vi "Dresden R2R Sputter 03.02.2018 IY24.vi"() -> ()   [LabVIEW 2009] (continued)
                              }
                              frame #1 {
                              }
                            }
                          }
                        }
                      }
                      frame #1 {
                      }
                    }
                  }
                  frame #1 {
                  }
                }
              }
              frame #1 {
              }
            }
          }
          frame #3 {
            # "STARTED UP CH2"
            n11092 = disable-structure shown="Disabled" {
              frame #0 {
                n11093 = local read "Semi"() -> (w17910:bool)
                n11094 = case shown="False" w17910 {
                  frame #0 {
                    n11095 = local read "started_up_ch2"() -> (w17911:bool)
                    n11096 = case shown="False" w17911 {
                      frame #0 {
                        n11097 = stacked-sequence {
                          frame #0 {
                            n11098 = local read "Semi"() -> (w17912:bool)
                            n11099 = case shown="False" w17912 {
                              frame #0 {
                                n11100 = local write "Start_up_ch2"(TRUE ("Start_up_ch2")) -> ()
                              }
                              frame #1 {
                              }
                            }
                          }
                          frame #1 {
                            n11101 = local read "Semi"() -> (w17914:bool)
                            n11102 = case shown="False" w17914 {
                              frame #0 {
                                n11103 = Wait (ms)(milliseconds to wait=u32 18000) -> ()  [unwired: 1 out]
                              }
                              frame #1 {
                              }
                            }
                          }
                          frame #2 {
                            n11104 = local read "Semi"() -> (w17916:bool)
                            n11105 = case shown="False" w17916 {
                              frame #0 {
                                n11106 = while {
                                i -> [w17921]
                                stop <- w17918 stop-if-true
                                n11107 = Greater?(x=w17921, y=90) -> (0:w17919:bool)
                                n11108 = local read "started_up_ch2"() -> (w17917:bool)
                                n11109 = case shown="True" w17919 {
                                frame #0 {
                                }
                                frame #1 {
                                n11110 = local write "Semi"(TRUE ("Semi")) -> ()
                                n11111 = local write "Error Message"("Chamber 2 Pressure is not suitable  \nfor transfer process!\nPlease check connections." ("Error Message")) -> ()
                                }
                                }
                                n11112 = case shown="False" w17917 {
                                tunnel: [FALSE TRUE] -> w17918
                                frame #0 {
                                n11113 = Wait Until Next ms Multiple(millisecond multiple=u32 200) -> ()  [unwired: 1 out]
                                }
                                frame #1 {
                                }
                                }
                                }
                              }
                              frame #1 {
                              }
                            }
                          }
                          frame #3 {
                            n11114 = local read "Semi"() -> (w17927:bool)
                            n11115 = case shown="False" w17927 {
                              frame #0 {
                                n11116 = local write "CH1_2_trns_1"(TRUE ("CH1_2_trns_0")) -> ()
                                n11117 = Wait (ms)(milliseconds to wait=u32 1000) -> ()  [unwired: 1 out]
                              }
                              frame #1 {
                              }
                            }
                          }
                        }
                      }
                      frame #1 {
                      }
                    }
                  }
                  frame #1 {
                  }
                }
              }
              frame #1 {
              }
            }
          }
          frame #4 {
            # "TRNS GV OPEN"
            n11118 = local read "Semi"() -> (w17930:bool)
            n11119 = case shown="False" w17930 {
              frame #0 {
                n11120 = stacked-sequence {
                  frame #0 {
                    n11121 = local read "Semi"() -> (w17931:bool)
                    n11122 = case shown="False" w17931 {
                      frame #0 {
                        n11123 = while {
                          i -> [w17938]
                          stop <- w17933 stop-if-true
                          n11124 = Greater?(x=w17938, y=50) -> (0:w17936:bool)
                          n11125 = local read "Ch1_Trns_gv_bp2_di"() -> (w17932:bool)
                          n11126 = case shown="True" w17936 {
                            frame #0 {
                            }
                            frame #1 {
                              n11127 = local write "Semi"(TRUE ("Semi")) -> ()
                              n11128 = local write "Error Message"("Transfer process was cancelled.\nPlease check CH1-Trns-GV connections." ("Error Message")) -> ()
                            }
                          }
                          n11129 = case shown="False" w17932 {
                            tunnel: [FALSE TRUE] -> w17935
                            frame #0 {
                              n11130 = Wait Until Next ms Multiple(millisecond multiple=u32 200) -> ()  [unwired: 1 out]
                              n11131 = local write "Ch1_Trns_gv_bp2_do"(TRUE ("Ch1_pet_cool_up_do")) -> ()
                            }
                            frame #1 {
                            }
                          }
                          n11132 = local read "Semi"() -> (w17934:bool)
                          n11133 = Or(x=w17935, y=w17934) -> (x .or. y?=w17933:bool)
                        }
                      }
                      frame #1 {
                      }
                    }
                  }
                  frame #1 {
                    n11134 = local read "Semi"() -> (w17945:bool)
                    n11135 = case shown="False" w17945 {
                      frame #0 {
                        n11136 = Wait (ms)(milliseconds to wait=u32 500) -> ()  [unwired: 1 out]
                      }
                      frame #1 {
                      }
                    }
                  }
                  frame #2 {
                    n11137 = local read "Semi"() -> (w17947:bool)
                    n11138 = case shown="False" w17947 {
                      frame #0 {
                        n11139 = while {
                          i -> [w17954]
                          stop <- w17949 stop-if-true
                          n11140 = Greater?(x=w17954, y=50) -> (0:w17952:bool)
                          n11141 = local read "Ch2_trns_gv_bp_di"() -> (w17948:bool)
                          n11142 = case shown="True" w17952 {
                            frame #0 {
                            }
                            frame #1 {
                              n11143 = local write "Semi"(TRUE ("Semi")) -> ()
                              n11144 = local write "Error Message"("Transfer process was cancelled.\nPlease check CH1-Trns-GV connections." ("Error Message")) -> ()
                            }
                          }
                          n11145 = case shown="False" w17948 {
                            tunnel: [FALSE TRUE] -> w17951
                            frame #0 {
                              n11146 = Wait Until Next ms Multiple(millisecond multiple=u32 200) -> ()  [unwired: 1 out]
                              n11147 = local write "Ch2_trns_gv_bp_do"(TRUE ("Ch1_pet_cool_up_do")) -> ()
                            }
                            frame #1 {
                            }
                          }
                          n11148 = local read "Semi"() -> (w17950:bool)
                          n11149 = Or(x=w17951, y=w17950) -> (x .or. y?=w17949:bool)
                        }
                      }
                      frame #1 {
                      }
                    }
                  }
                  frame #3 {
                    n11150 = local read "Semi"() -> (w17961:bool)
                    n11151 = case shown="False" w17961 {
                      frame #0 {
                        n11152 = Wait (ms)(milliseconds to wait=u32 500) -> ()  [unwired: 1 out]
                      }
                      frame #1 {
                      }
                    }
                  }
                }
              }
              frame #1 {
              }
            }
          }
          frame #5 {
            # "TRNS GV OPEN"
            n11153 = local read "Semi"() -> (w17963:bool)
            n11154 = case shown="False" w17963 {
              frame #0 {
                n11155 = stacked-sequence {
                  frame #0 {
                    n11156 = local read "Semi"() -> (w17964:bool)
                    n11157 = case shown="False" w17964 {
                      frame #0 {
                        n11158 = local write "Ch1_Trns_gv_close_do"(FALSE ("Ch1_pet_cool_up_do")) -> ()
                      }
                      frame #1 {
                      }
                    }
                  }
                  frame #1 {
                    n11159 = local read "Semi"() -> (w17966:bool)
                    n11160 = case shown="False" w17966 {
                      frame #0 {
                        n11161 = while {
                          i -> [w17973]
                          stop <- w17968 stop-if-true
                          n11162 = Greater?(x=w17973, y=500) -> (0:w17971:bool)
                          n11163 = local read "Ch1_Trns_gv_open_di"() -> (w17967:bool)
                          n11164 = case shown="True" w17971 {
                            frame #0 {
                            }
                            frame #1 {
                              n11165 = local write "Semi"(TRUE ("Semi")) -> ()
                              n11166 = local write "Error Message"("Transfer process was cancelled.\nPlease check CH1-Trns-GV connections." ("Error Message")) -> ()
                            }
                          }
                          n11167 = case shown="False" w17967 {
                            tunnel: [FALSE TRUE] -> w17970
                            frame #0 {
                              n11168 = Wait Until Next ms Multiple(millisecond multiple=u32 200) -> ()  [unwired: 1 out]
                              n11169 = local write "Ch1_Trns_gv_open_do"(TRUE ("Ch1_pet_cool_up_do")) -> ()
                            }
                            frame #1 {
                            }
                          }
                          n11170 = local read "Semi"() -> (w17969:bool)
                          n11171 = Or(x=w17970, y=w17969) -> (x .or. y?=w17968:bool)
                        }
                      }
                      frame #1 {
                      }
                    }
                  }
                  frame #2 {
                    n11172 = local read "Semi"() -> (w17980:bool)
                    n11173 = case shown="False" w17980 {
                      frame #0 {
                        n11174 = local write "CH1_2trns_2"(TRUE ("CH1_2trns_5")) -> ()
                        n11175 = Wait (ms)(milliseconds to wait=u32 500) -> ()  [unwired: 1 out]
                      }
                      frame #1 {
                      }
                    }
                  }
                }
              }
              frame #1 {
              }
            }
          }
          frame #6 {
            # "TRNS GV control Trnsgv 2_3"
            n11176 = local read "Semi"() -> (w17983:bool)
            n11177 = case shown="False" w17983 {
              frame #0 {
                n11178 = stacked-sequence {
                  frame #0 {
                    n11179 = local read "Semi"() -> (w17984:bool)
                    n11180 = case shown="False" w17984 {
                      frame #0 {
                        n11181 = while {
                          i -> [w17991]
                          stop <- w17986 stop-if-true
                          n11182 = Greater?(x=w17991, y=50) -> (0:w17989:bool)
                          n11183 = local read "Ch1_TGV_control_di"() -> (w17985:bool)
                          n11184 = case shown="True" w17989 {
                            frame #0 {
                            }
                            frame #1 {
                              n11185 = local write "Semi"(TRUE ("Semi")) -> ()
                              n11186 = local write "Error Message"("Transfer process was cancelled.\nPlease check TRNS-GV connections." ("Error Message")) -> ()
                            }
                          }
                          n11187 = case shown="True" w17985 {
                            tunnel: [TRUE FALSE] -> w17988
                            frame #0 {
                            }
                            frame #1 {
                              n11188 = Wait Until Next ms Multiple(millisecond multiple=u32 200) -> ()  [unwired: 1 out]
                              n11189 = local write "Ch1_TGV_control_do"(FALSE ("Ch1_pet_cool_up_do")) -> ()
                            }
                          }
                          n11190 = local read "Semi"() -> (w17987:bool)
                          n11191 = Or(x=w17988, y=w17987) -> (x .or. y?=w17986:bool)
                        }
                      }
                      frame #1 {
                      }
                    }
                  }
                  frame #1 {
                    n11192 = local read "Semi"() -> (w17998:bool)
                    n11193 = case shown="False" w17998 {
                      frame #0 {
                        n11194 = local write "CH1_2trns_3"(TRUE ("CH1_2trns_5")) -> ()
                        n11195 = Wait (ms)(milliseconds to wait=u32 500) -> ()  [unwired: 1 out]
                      }
                      frame #1 {
                      }
                    }
                  }
                }
              }
              frame #1 {
              }
            }
          }
          frame #7 {
            # "TRNS GV control Trnsgv 2_3"
            n11196 = local read "Semi"() -> (w18001:bool)
            n11197 = case shown="False" w18001 {
              frame #0 {
                n11198 = stacked-sequence {
                  frame #0 {
                    n11199 = local read "Semi"() -> (w18002:bool)
                    n11200 = case shown="False" w18002 {
                      frame #0 {
                        n11201 = while {
                          i -> [w18009]
                          stop <- w18004 stop-if-true
                          n11202 = Greater?(x=w18009, y=50) -> (0:w18007:bool)
                          n11203 = local read "Ch2_Trns_interlock_di"() -> (w18003:bool)
                          n11204 = case shown="True" w18007 {
                            frame #0 {
                            }
                            frame #1 {
                              n11205 = local write "Semi"(TRUE ("Semi")) -> ()
                              n11206 = local write "Error Message"("Transfer process was cancelled.\nPlease check TRNS-GV connections." ("Error Message")) -> ()
                            }
                          }
                          n11207 = case shown="False" w18003 {
                            tunnel: [w18011 TRUE] -> w18006
                            frame #0 {
                              n11208 = local read "Ch2_TGV_control_di"() -> (w18010:bool)
                              n11209 = case shown="False" w18010 {
                                tunnel: [FALSE TRUE] -> w18011
                                frame #0 {
                                n11210 = Wait Until Next ms Multiple(millisecond multiple=u32 200) -> ()  [unwired: 1 out]
                                n11211 = local write "Ch2_TGV_control_do"(TRUE ("Ch1_pet_cool_up_do")) -> ()
                                }
                                frame #1 {
                                }
                              }
                            }
                            frame #1 {
                            }
                          }
                          n11212 = local read "Semi"() -> (w18005:bool)
                          n11213 = Or(x=w18006, y=w18005) -> (x .or. y?=w18004:bool)
                        }
                      }
                      frame #1 {
                      }
                    }
                  }
                  frame #1 {
                    n11214 = local read "Semi"() -> (w18019:bool)
                    n11215 = case shown="False" w18019 {
                      frame #0 {
                        n11216 = local write "CH1_2trns_3"(TRUE ("CH1_2trns_5")) -> ()
                        n11217 = Wait (ms)(milliseconds to wait=u32 500) -> ()  [unwired: 1 out]
                      }
                      frame #1 {
                      }
                    }
                  }
                }
              }
              frame #1 {
              }
            }
          }
          frame #8 {
            # "TRNS GV control Trnsgv 3_4"
            n11218 = local read "Semi"() -> (w18022:bool)
            n11219 = case shown="False" w18022 {
              frame #0 {
                n11220 = stacked-sequence {
                  frame #0 {
                    n11221 = local read "Semi"() -> (w18023:bool)
                    n11222 = case shown="False" w18023 {
                      frame #0 {
                        n11223 = while {
                          i -> [w18030]
                          stop <- w18025 stop-if-true
                          n11224 = Greater?(x=w18030, y=50) -> (0:w18028:bool)
                          n11225 = local read "Ch3_Trns_interlock_di"() -> (w18024:bool)
                          n11226 = case shown="True" w18028 {
                            frame #0 {
                            }
                            frame #1 {
                              n11227 = local write "Semi"(TRUE ("Semi")) -> ()
                              n11228 = local write "Error Message"("Transfer process was cancelled.\nPlease check TRNS-GV connections." ("Error Message")) -> ()
                            }
                          }
                          n11229 = case shown="False" w18024 {
                            tunnel: [w18032 TRUE] -> w18027
                            frame #0 {
                              n11230 = local read "Ch3_TGV_control_di"() -> (w18031:bool)
                              n11231 = case shown="False" w18031 {
                                tunnel: [FALSE TRUE] -> w18032
                                frame #0 {
                                n11232 = Wait Until Next ms Multiple(millisecond multiple=u32 200) -> ()  [unwired: 1 out]
                                n11233 = local write "Ch3_TGV_control_do"(TRUE ("Ch1_pet_cool_up_do")) -> ()
                                }
                                frame #1 {
                                }
                              }
                            }
                            frame #1 {
                            }
                          }
                          n11234 = local read "Semi"() -> (w18026:bool)
                          n11235 = Or(x=w18027, y=w18026) -> (x .or. y?=w18025:bool)
                        }
                      }
                      frame #1 {
                      }
                    }
                  }
                  frame #1 {
                    n11236 = local read "Semi"() -> (w18040:bool)
                    n11237 = case shown="False" w18040 {
                      frame #0 {
                        n11238 = local write "CH1_2trns_4"(TRUE ("CH1_2trns_5")) -> ()
                        n11239 = Wait (ms)(milliseconds to wait=u32 500) -> ()  [unwired: 1 out]
                      }
                      frame #1 {
                      }
                    }
                  }
                }
              }
              frame #1 {
              }
            }
          }
          frame #9 {
            # "Right slow deactive"
            n11240 = local read "Semi"() -> (w18043:bool)
            n11241 = case shown="False" w18043 {
              frame #0 {
                n11242 = stacked-sequence {
                  frame #0 {
                    n11243 = local read "Semi"() -> (w18044:bool)
                    n11244 = case shown="False" w18044 {
                      frame #0 {
                        n11245 = while {
                          i -> [w18047]
                          stop <- w18048 stop-if-true
                          n11246 = Greater?(x=w18047, y=50) -> (0:w18045:bool)
                          n11247 = local read "Cnt_Right_slow_di"() -> (w18051:bool)
                          n11248 = case shown="True" w18045 {
                            frame #0 {
                            }
                            frame #1 {
                              n11249 = local write "Semi"(TRUE ("Semi")) -> ()
                              n11250 = local write "Error Message"("Transfer process was\ncancelled.Please check right slow sensor." ("Error Message")) -> ()
                            }
                          }
                          n11251 = case shown="False" w18051 {
                            tunnel: [FALSE ("Ch1_pet_cool_up_do") TRUE ("Ch1_pet_cool_up_do")] -> w18050
                            frame #0 {
                              n11252 = Wait Until Next ms Multiple(millisecond multiple=u32 200) -> ()  [unwired: 1 out]
                              n11253 = local write "Cnt_Right_slow_do"(TRUE ("Ch1_pet_cool_up_do")) -> ()
                            }
                            frame #1 {
                            }
                          }
                          n11254 = local read "Semi"() -> (w18049:bool)
                          n11255 = Or(x=w18050, y=w18049) -> (x .or. y?=w18048:bool)
                        }
                      }
                      frame #1 {
                      }
                    }
                  }
                  frame #1 {
                    n11256 = local read "Semi"() -> (w18058:bool)
                    n11257 = case shown="False" w18058 {
                      frame #0 {
                        n11258 = local write "CH1_2trns_5"(TRUE ("CH1_2trns_7")) -> ()
                        n11259 = Wait (ms)(milliseconds to wait=u32 500) -> ()  [unwired: 1 out]
                      }
                      frame #1 {
                      }
                    }
                  }
                }
              }
              frame #1 {
              }
            }
          }
          frame #10 {
            # "Right limit deactive"
            n11260 = local read "Semi"() -> (w18061:bool)
            n11261 = case shown="False" w18061 {
              frame #0 {
                n11262 = stacked-sequence {
                  frame #0 {
                    n11263 = local read "Semi"() -> (w18062:bool)
                    n11264 = case shown="False" w18062 {
                      frame #0 {
                        n11265 = while {
                          i -> [w18063]
                          stop <- w18067 stop-if-true
                          n11266 = Greater?(x=w18063, y=50) -> (0:w18065:bool)
                          n11267 = local read "Cnt_Right_limit_di"() -> (w18069:bool)
                          n11268 = case shown="True" w18065 {
                            frame #0 {
                            }
                            frame #1 {
                              n11269 = local write "Semi"(TRUE ("Semi")) -> ()
                              n11270 = local write "Error Message"("Transfer process was\ncancelled.Please check right limit sensor." ("Error Message")) -> ()
                            }
                          }
                          n11271 = case shown="False" w18069 {
                            tunnel: [FALSE ("Ch1_pet_cool_up_do") TRUE ("Ch1_pet_cool_up_do")] -> w18068
                            frame #0 {
                              n11272 = Wait Until Next ms Multiple(millisecond multiple=u32 200) -> ()  [unwired: 1 out]
                              n11273 = local write "Cnt_Right_limit_do"(TRUE ("Ch1_pet_cool_up_do")) -> ()
                            }
                            frame #1 {
                            }
                          }
                          n11274 = local read "Semi"() -> (w18066:bool)
                          n11275 = Or(x=w18068, y=w18066) -> (x .or. y?=w18067:bool)
                        }
                      }
                      frame #1 {
                      }
                    }
                  }
                  frame #1 {
                    n11276 = local read "Semi"() -> (w18076:bool)
                    n11277 = case shown="False" w18076 {
                      frame #0 {
                        n11278 = local write "CH1_2trns_6"(TRUE ("CH1_2trns_7")) -> ()
                        n11279 = Wait (ms)(milliseconds to wait=u32 500) -> ()  [unwired: 1 out]
                      }
                      frame #1 {
                      }
                    }
                  }
                }
              }
              frame #1 {
              }
            }
          }
          frame #11 {
            # "Left slow active"
            n11280 = local read "Semi"() -> (w18079:bool)
            n11281 = case shown="False" w18079 {
              frame #0 {
                n11282 = stacked-sequence {
                  frame #0 {
                    n11283 = local read "Semi"() -> (w18080:bool)
                    n11284 = case shown="False" w18080 {
                      frame #0 {
                        n11285 = while {
                          i -> [w18081]
                          stop <- w18085 stop-if-true
                          n11286 = Greater?(x=w18081, y=50) -> (0:w18083:bool)
                          n11287 = local read "Cnt_Left_slow_di"() -> (w18087:bool)
                          n11288 = case shown="True" w18083 {
                            frame #0 {
                            }
                            frame #1 {
                              n11289 = local write "Semi"(TRUE ("Semi")) -> ()
                              n11290 = local write "Error Message"("Transfer process was\ncancelled.Please check left slow sensor." ("Error Message")) -> ()
                            }
                          }
                          n11291 = case shown="True" w18087 {
                            tunnel: [TRUE ("Ch1_pet_cool_up_do") FALSE ("Ch1_pet_cool_up_do")] -> w18086
                            frame #0 {
                            }
                            frame #1 {
                              n11292 = Wait Until Next ms Multiple(millisecond multiple=u32 200) -> ()  [unwired: 1 out]
                              n11293 = local write "Cnt_Left_slow_do"(FALSE ("Ch1_pet_cool_up_do")) -> ()
                            }
                          }
                          n11294 = local read "Semi"() -> (w18084:bool)
                          n11295 = Or(x=w18086, y=w18084) -> (x .or. y?=w18085:bool)
                        }
                      }
                      frame #1 {
                      }
                    }
                  }
                  frame #1 {
                    n11296 = local read "Semi"() -> (w18094:bool)
                    n11297 = case shown="False" w18094 {
                      frame #0 {
                        n11298 = local write "CH1_2trns_7"(TRUE ("CH1_2trns_6b")) -> ()
                        n11299 = Wait (ms)(milliseconds to wait=u32 500) -> ()  [unwired: 1 out]
                      }
                      frame #1 {
                      }
                    }
                  }
                }
              }
              frame #1 {
              }
            }
          }
          frame #12 {
            # "Left limit active"
            n11300 = local read "Semi"() -> (w18097:bool)
            n11301 = case shown="False" w18097 {
              frame #0 {
                n11302 = stacked-sequence {
                  frame #0 {
                    n11303 = local read "Semi"() -> (w18098:bool)
                    n11304 = case shown="False" w18098 {
                      frame #0 {
                        n11305 = while {
                          i -> [w18099]
                          stop <- w18103 stop-if-true
                          n11306 = Greater?(x=w18099, y=50) -> (0:w18101:bool)
                          n11307 = local read "Cnt_Left_limit_di"() -> (w18105:bool)
                          n11308 = case shown="True" w18101 {
                            frame #0 {
                            }
                            frame #1 {
                              n11309 = local write "Semi"(TRUE ("Semi")) -> ()
                              n11310 = local write "Error Message"("Transfer process was\ncancelled.Please check left limit sensor." ("Error Message")) -> ()
                            }
                          }
                          n11311 = case shown="True" w18105 {
                            tunnel: [TRUE ("Ch1_pet_cool_up_do") FALSE ("Ch1_pet_cool_up_do")] -> w18104
                            frame #0 {
                            }
                            frame #1 {
                              n11312 = Wait Until Next ms Multiple(millisecond multiple=u32 200) -> ()  [unwired: 1 out]
                              n11313 = local write "Cnt_Left_limit_do"(FALSE ("Ch1_pet_cool_up_do")) -> ()
                            }
                          }
                          n11314 = local read "Semi"() -> (w18102:bool)
                          n11315 = Or(x=w18104, y=w18102) -> (x .or. y?=w18103:bool)
                        }
                      }
                      frame #1 {
                      }
                    }
                  }
                  frame #1 {
                    n11316 = local read "Semi"() -> (w18112:bool)
                    n11317 = case shown="False" w18112 {
                      frame #0 {
                        n11318 = local write "CH1_2trns_8"(TRUE ("CH1_2trns_6c")) -> ()
                        n11319 = Wait (ms)(milliseconds to wait=u32 500) -> ()  [unwired: 1 out]
                      }
                      frame #1 {
                      }
                    }
                  }
                }
              }
              frame #1 {
              }
            }
          }
          frame #13 {
            # "Casette Direction"
            n11320 = local read "Semi"() -> (w18115:bool)
            n11321 = case shown="False" w18115 {
              frame #0 {
                n11322 = stacked-sequence {
                  frame #0 {
                    n11323 = local read "Semi"() -> (w18116:bool)
                    n11324 = case shown="False" w18116 {
                      frame #0 {
                        n11325 = while {
                          i -> [w18122]
                          stop <- w18117 stop-if-true
                          n11326 = Greater?(x=w18122, y=50) -> (0:w18123:bool)
                          n11327 = case shown="True" w18123 {
                            frame #0 {
                            }
                            frame #1 {
                              n11328 = local write "Semi"(TRUE ("Semi")) -> ()
                              n11329 = local write "Error Message"("Transfer process was cancelled.\nPlease check Casette Direction connections." ("Error Message")) -> ()
                            }
                          }
                          n11330 = local read "Casette_servo_left_direction_di"() -> (w18120:bool)
                          n11331 = case shown="False" w18120 {
                            tunnel: [FALSE ("Casette_servo_left_direction_do") TRUE ("Casette_servo_left_direction_do")] -> w18119
                            frame #0 {
                              n11332 = Wait Until Next ms Multiple(millisecond multiple=u32 200) -> ()  [unwired: 1 out]
                              n11333 = local write "Casette_servo_left_direction_do"(TRUE ("Casette_servo_left_direction_do")) -> ()
                            }
                            frame #1 {
                            }
                          }
                          n11334 = local read "Semi"() -> (w18118:bool)
                          n11335 = Or(x=w18119, y=w18118) -> (x .or. y?=w18117:bool)
                        }
                      }
                      frame #1 {
                      }
                    }
                  }
                  frame #1 {
                    n11336 = local read "Semi"() -> (w18130:bool)
                    n11337 = case shown="False" w18130 {
                      frame #0 {
                        n11338 = local write "CH1_2trns_9"(TRUE ("CH1_2trns_7")) -> ()
                        n11339 = Wait (ms)(milliseconds to wait=u32 500) -> ()  [unwired: 1 out]
                      }
                      frame #1 {
                      }
                    }
                  }
                }
              }
              frame #1 {
              }
            }
          }
          frame #14 {
            # "SET CASSETTE SERVO  SPEED 300"
            n11340 = local read "Semi"() -> (w18133:bool)
            n11341 = case shown="False" w18133 {
              frame #0 {
                n11342 = stacked-sequence {
                  frame #0 {
                    n11343 = local read "Semi"() -> (w18134:bool)
                    n11344 = case shown="False" w18134 {
                      frame #0 {
                        n11345 = local write "Cassette_servo_speed_value"(u16 300 ("Cassette_servo_speed_value")) -> ()
                      }
                      frame #1 {
                      }
                    }
                  }
                  frame #1 {
                    n11346 = local read "Semi"() -> (w18136:bool)
                    n11347 = case shown="False" w18136 {
                      frame #0 {
                        n11348 = Wait (ms)(milliseconds to wait=u32 200) -> ()  [unwired: 1 out]
                      }
                      frame #1 {
                      }
                    }
                  }
                  frame #2 {
                    n11349 = local read "Semi"() -> (w18138:bool)
                    n11350 = case shown="False" w18138 {
                      frame #0 {
                        n11351 = local write "Cassette_servo_speed_auto_set"(TRUE ("Cassette_servo_speed_set")) -> ()
                      }
                      frame #1 {
                      }
                    }
                  }
                  frame #3 {
                    n11352 = local read "Semi"() -> (w18140:bool)
                    n11353 = case shown="False" w18140 {
                      frame #0 {
                        n11354 = Wait (ms)(milliseconds to wait=u32 200) -> ()  [unwired: 1 out]
                      }
                      frame #1 {
                      }
                    }
                  }
                  frame #4 {
                    n11355 = local read "Semi"() -> (w18142:bool)
                    n11356 = case shown="False" w18142 {
                      frame #0 {
                        n11357 = local write "CH1_2trns_10"(TRUE ("CH1_2trns_7")) -> ()
                        n11358 = Wait (ms)(milliseconds to wait=u32 500) -> ()  [unwired: 1 out]
                      }
                      frame #1 {
                      }
                    }
                  }
                }
              }
              frame #1 {
              }
            }
          }
          frame #15 {
            # "Casette Servo Start"
            n11359 = local read "Semi"() -> (w18145:bool)
            n11360 = case shown="False" w18145 {
              frame #0 {
                n11361 = stacked-sequence {
                  frame #0 {
                    n11362 = while {
                      i -> [w18151]
                      stop <- w18146 stop-if-true
                      n11363 = Greater?(x=w18151, y=50) -> (0:w18152:bool)
                      n11364 = local read "Casette_servo_start/stop_di"() -> (w18149:bool)
                      n11365 = case shown="True" w18152 {
                        frame #0 {
                        }
                        frame #1 {
                          n11366 = local write "Semi"(TRUE ("Semi")) -> ()
                          n11367 = local write "Error Message"("Transfer process was cancelled.\nPlease check Casette connections." ("Error Message")) -> ()
                        }
                      }
                      n11368 = case shown="False" w18149 {
                        tunnel: [FALSE ("Casette_servo_left_direction_do") TRUE ("Casette_servo_left_direction_do")] -> w18148
                        frame #0 {
                          n11369 = Wait Until Next ms Multiple(millisecond multiple=u32 200) -> ()  [unwired: 1 out]
                          n11370 = local write "Casette_servo_start/stop_do"(TRUE ("Casette_servo_left_direction_do")) -> ()
                        }
                        frame #1 {
                        }
                      }
                      n11371 = local read "Semi"() -> (w18147:bool)
                      n11372 = Or(x=w18148, y=w18147) -> (x .or. y?=w18146:bool)
                    }
                  }
                  frame #1 {
                    n11373 = local read "Semi"() -> (w18159:bool)
                    n11374 = case shown="False" w18159 {
                      frame #0 {
                        n11375 = local write "CH1_2trns_11"(TRUE ("CH1_2trns_9")) -> ()
                        n11376 = Wait (ms)(milliseconds to wait=u32 500) -> ()  [unwired: 1 out]
                      }
                      frame #1 {
                      }
                    }
                  }
                }
              }
              frame #1 {
              }
            }
          }
          frame #16 {
            # "SET CASSETTE SERVO  SPEED 100"
            n11377 = local read "Semi"() -> (w18162:bool)
            n11378 = case shown="False" w18162 {
              frame #0 {
                n11379 = stacked-sequence {
                  frame #0 {
                    n11380 = while {
                      i -> [w18169]
                      stop <- w18165 stop-if-true
                      n11381 = local read "Ch2_Left_slow_di"() -> (w18163:bool)
                      n11382 = Greater?(x=w18169, y=1500) -> (0:w18168:bool)
                      n11383 = case shown="True" w18168 {
                        frame #0 {
                        }
                        frame #1 {
                          n11384 = local write "Semi"(TRUE ("Semi")) -> ()
                          n11385 = local write "Error Message"("Transfer process was cancelled.\nPlease check Casette & Sensor\nconnections." ("Error Message")) -> ()
                        }
                      }
                      n11386 = case shown="False" w18163 {
                        tunnel: [FALSE TRUE] -> w18166
                        frame #0 {
                          n11387 = Wait Until Next ms Multiple(millisecond multiple=u32 200) -> ()  [unwired: 1 out]
                        }
                        frame #1 {
                        }
                      }
                      n11388 = local read "Semi"() -> (w18164:bool)
                      n11389 = Or(x=w18166, y=w18164) -> (x .or. y?=w18165:bool)
                    }
                  }
                  frame #1 {
                    n11390 = disable-structure shown="Disabled" {
                      frame #0 {
                        n11391 = while {
                          i -> [w18184]
                          stop <- w18180 stop-if-true
                          n11392 = local read "Counter_read_data"() -> (w18177:i16)
                          n11393 = Greater?(x=w18184, y=5000) -> (0:w18183:bool)
                          n11394 = case shown="True" w18183 {
                            frame #0 {
                            }
                            frame #1 {
                              n11395 = local write "Semi"(TRUE ("Semi")) -> ()
                            }
                          }
                          n11396 = In Range and Coerce(upper limit=i16 1990, x=w18177, lower limit=i16 1980 ("upper limit")) -> (In Range?=w18175:bool)  [unwired: 1 out]
                          n11397 = case shown="True" w18175 {
                            tunnel: [FALSE TRUE] -> w18181
                            frame #0 {
                              n11398 = Wait Until Next ms Multiple(millisecond multiple=u32 200) -> ()  [unwired: 1 out]
                            }
                            frame #1 {
                            }
                          }
                          n11399 = local read "Semi"() -> (w18179:bool)
                          n11400 = Or(x=w18181, y=w18179) -> (x .or. y?=w18180:bool)
                        }
                      }
                      frame #1 {
                      }
                    }
                  }
                  frame #2 {
                    n11401 = local read "Semi"() -> (w18189:bool)
                    n11402 = case shown="False" w18189 {
                      frame #0 {
                        n11403 = local write "Cassette_servo_speed_value"(u16 100 ("Cassette_servo_speed_value")) -> ()
                      }
                      frame #1 {
                      }
                    }
                  }
                  frame #3 {
                    n11404 = local read "Semi"() -> (w18191:bool)
                    n11405 = case shown="False" w18191 {
                      frame #0 {
                        n11406 = Wait (ms)(milliseconds to wait=u32 200 ("millisecond multiple")) -> ()  [unwired: 1 out]
                      }
                      frame #1 {
                      }
                    }
                  }
                  frame #4 {
                    n11407 = local read "Semi"() -> (w18193:bool)
                    n11408 = case shown="False" w18193 {
                      frame #0 {
                        n11409 = local write "Cassette_servo_speed_auto_set"(TRUE ("Cassette_servo_speed_auto_set")) -> ()
                      }
                      frame #1 {
                      }
                    }
                  }
                  frame #5 {
                    n11410 = local read "Semi"() -> (w18195:bool)
                    n11411 = case shown="False" w18195 {
                      frame #0 {
                        n11412 = Wait (ms)(milliseconds to wait=u32 200 ("millisecond multiple")) -> ()  [unwired: 1 out]
                      }
                      frame #1 {
                      }
                    }
                  }
                  frame #6 {
                    n11413 = while {
                      i -> [w18200]
                      stop <- w18197 stop-if-true
                      n11414 = Greater?(x=w18200, y=50) -> (0:w18201:bool)
                      n11415 = local read "Cnt_Left_slow_di"() -> (w18203:bool)
                      n11416 = case shown="True" w18201 {
                        frame #0 {
                        }
                        frame #1 {
                          n11417 = local write "Semi"(TRUE ("Semi")) -> ()
                          n11418 = local write "Error Message"("\nPlease check connections." ("Error Message")) -> ()
                        }
                      }
                      n11419 = case shown="False" w18203 {
                        tunnel: [FALSE ("Cnt_Left_slow_do") TRUE ("Cnt_Left_slow_do")] -> w18199
                        frame #0 {
                          n11420 = Wait Until Next ms Multiple(millisecond multiple=u32 200) -> ()  [unwired: 1 out]
                          n11421 = local write "Cnt_Left_slow_do"(TRUE ("Cnt_Left_slow_do")) -> ()
                        }
                        frame #1 {
                        }